vi "01 Dryer_Performance_SM.vi"() -> ()   [LabVIEW 2012] (continued)
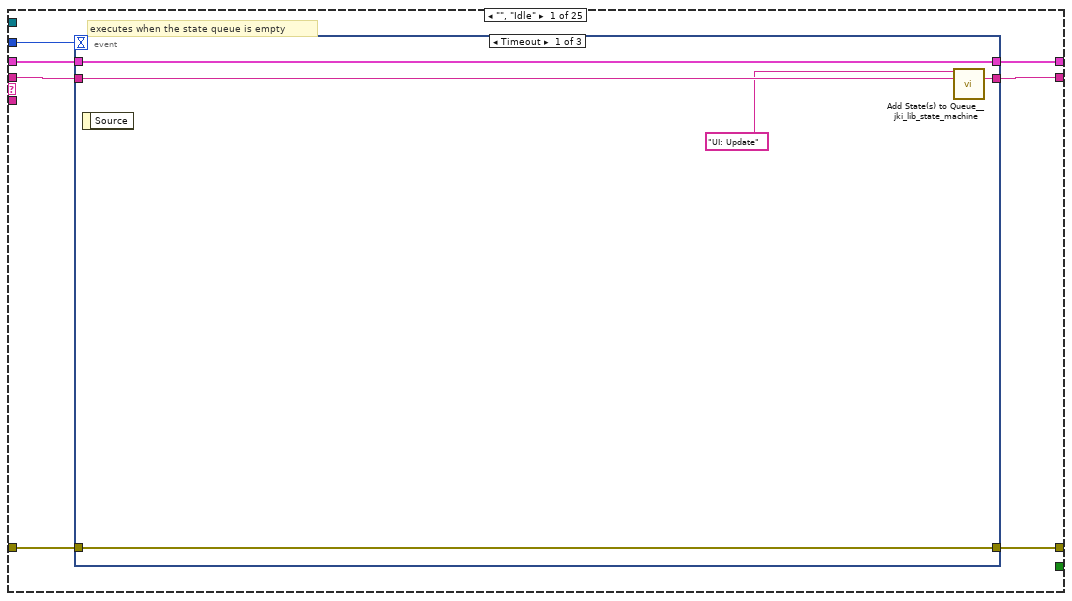
[diagram p3: hidden frame]
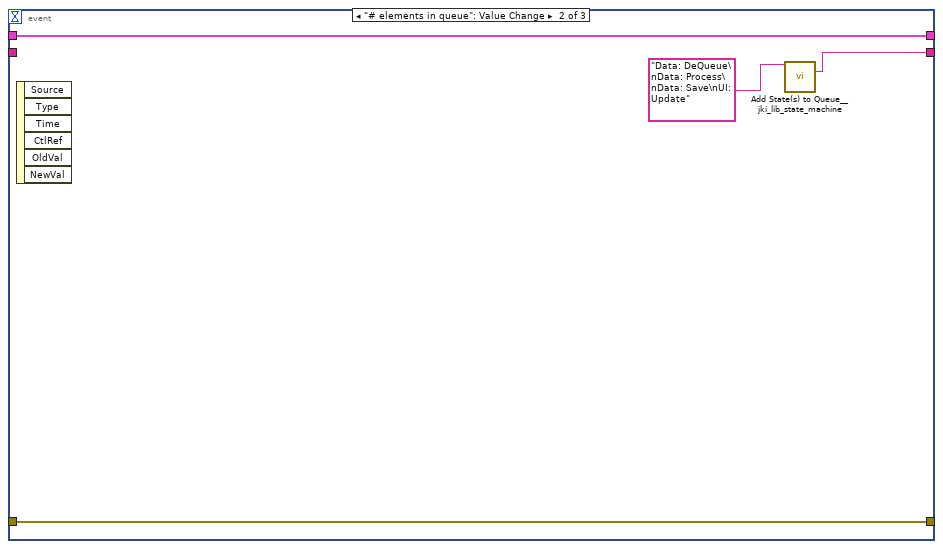
[diagram p4: hidden frame]
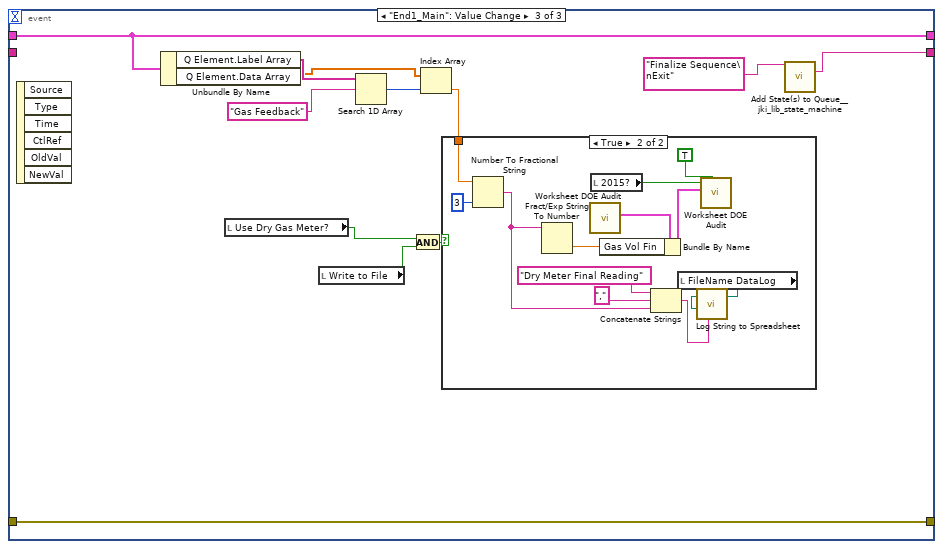
[diagram p5: hidden frame]
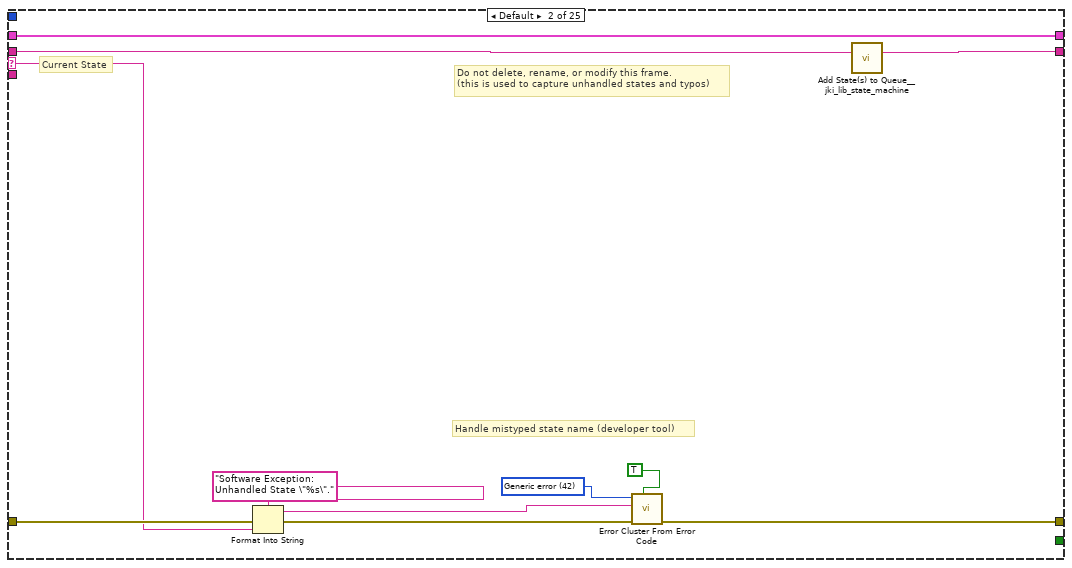
[diagram p7: hidden frame]
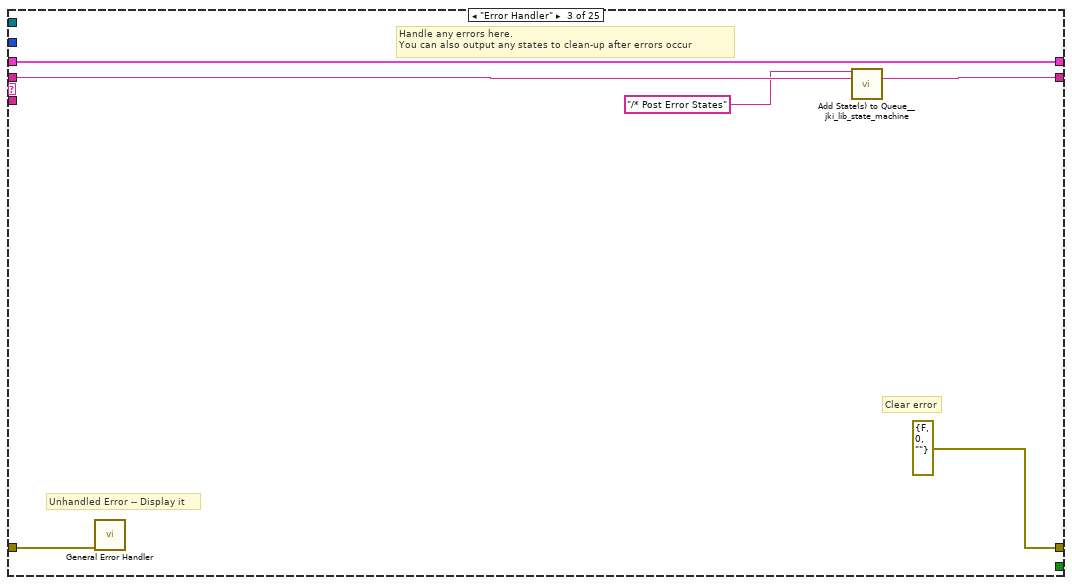
[diagram p8: hidden frame]
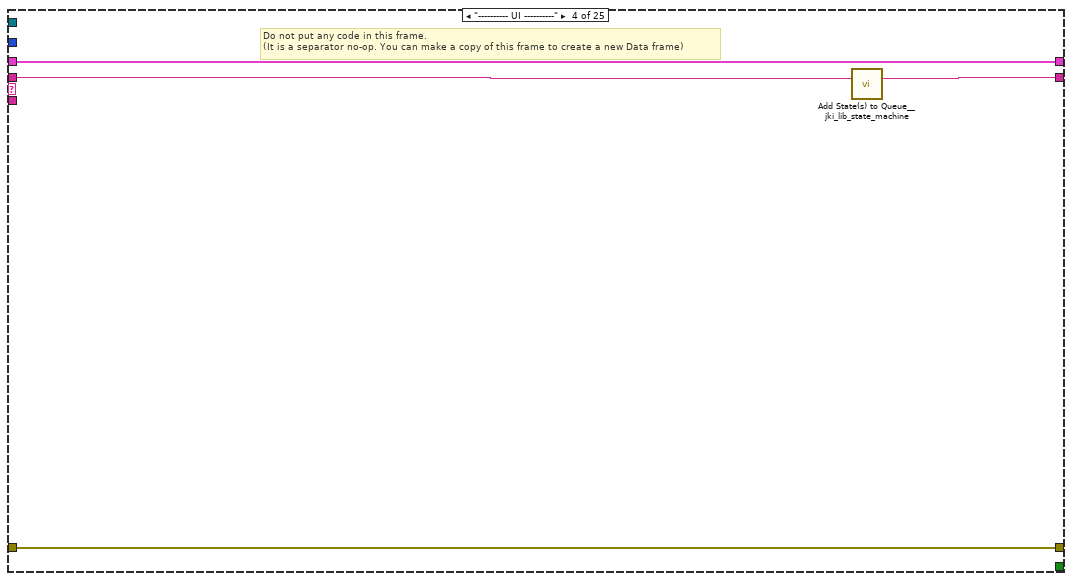
[diagram p9: hidden frame]
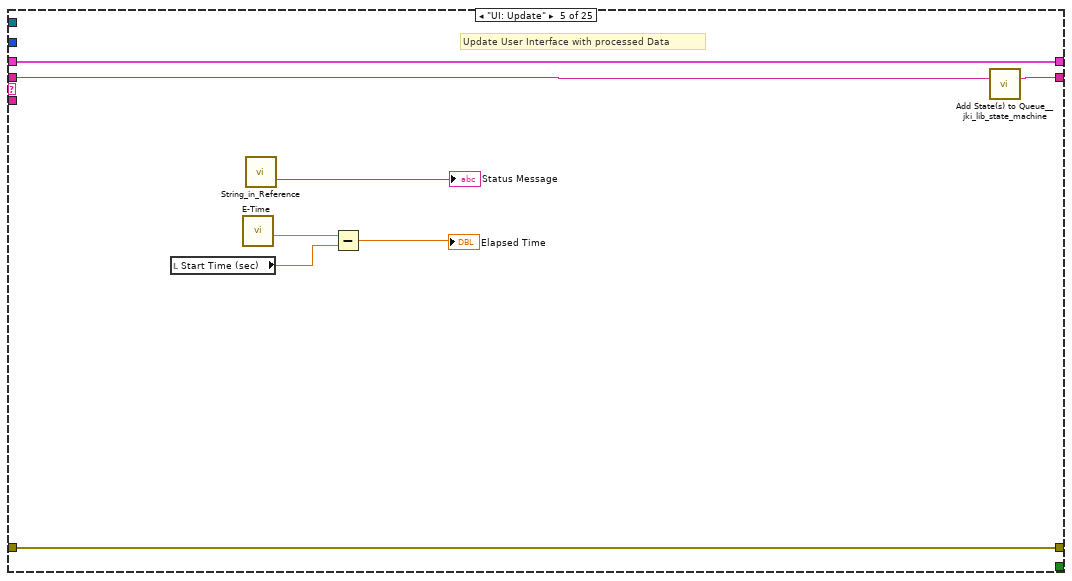
[diagram p10: hidden frame]
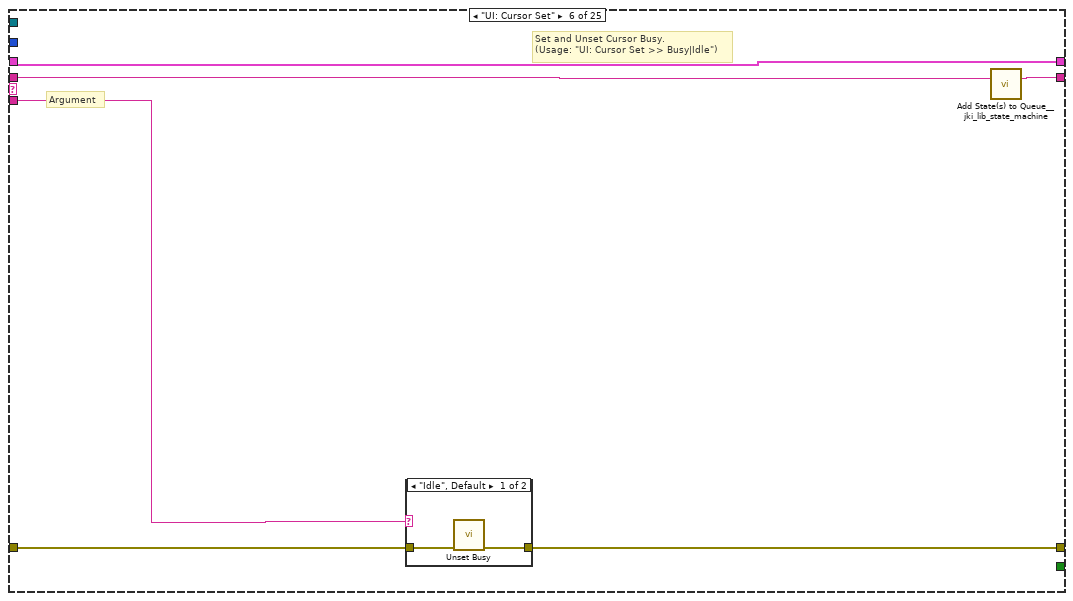
[diagram p11: hidden frame]
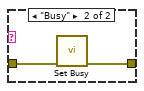
[diagram p12: hidden frame]
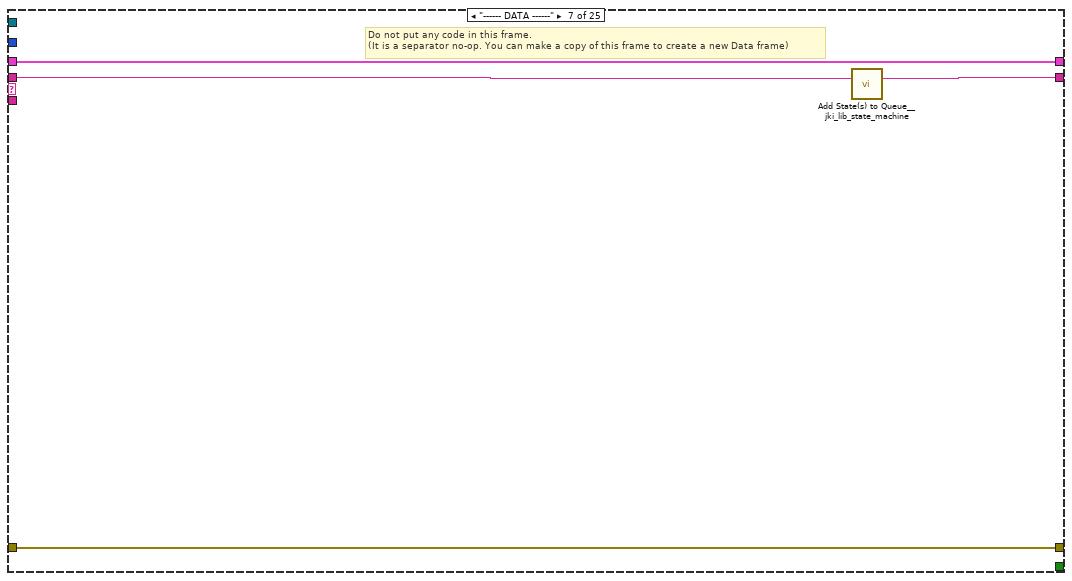
[diagram p13: hidden frame]
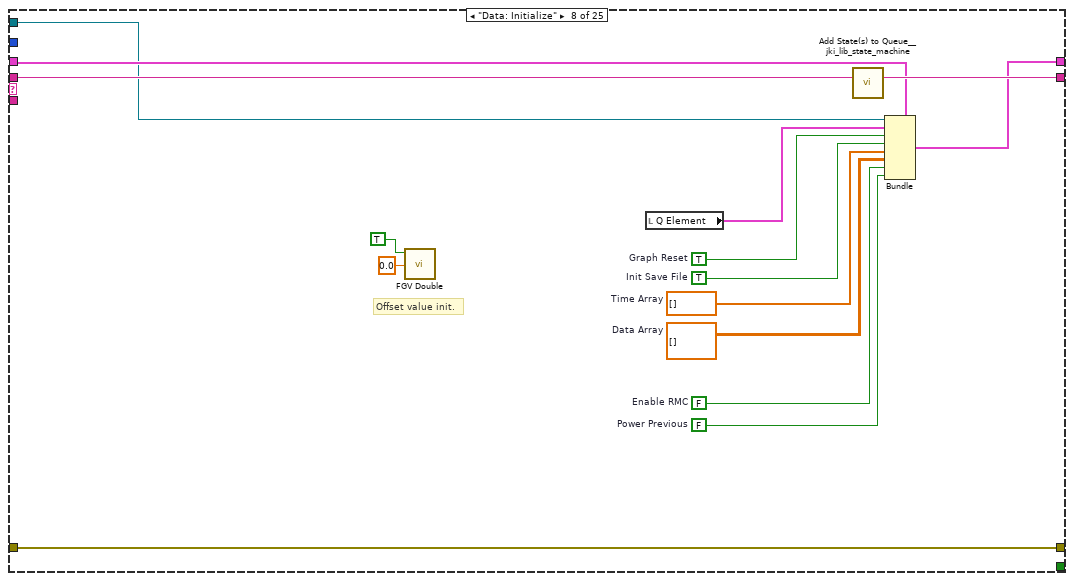
[diagram p14: hidden frame]
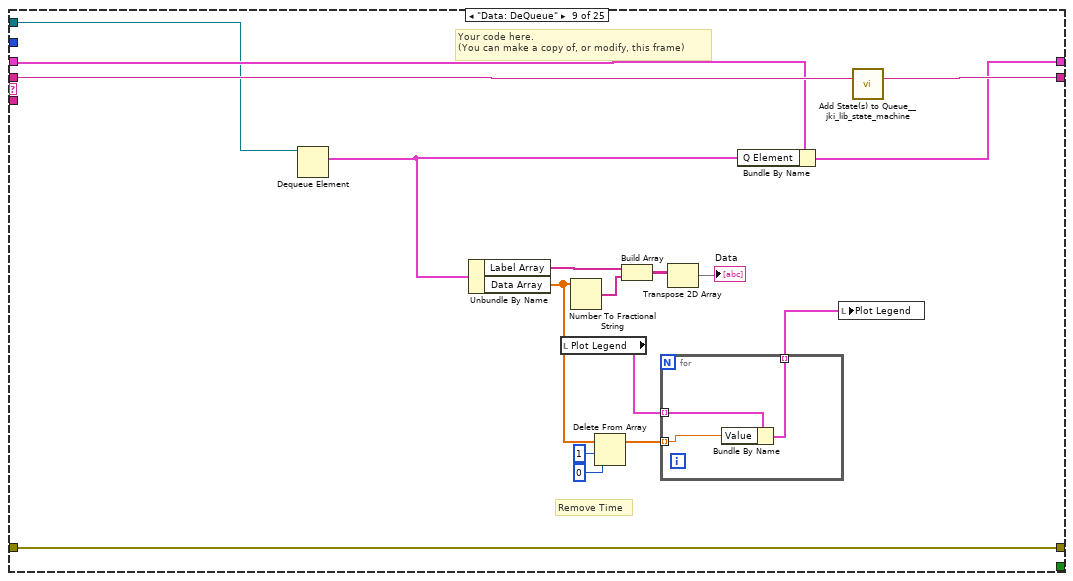
[diagram p15: hidden frame]
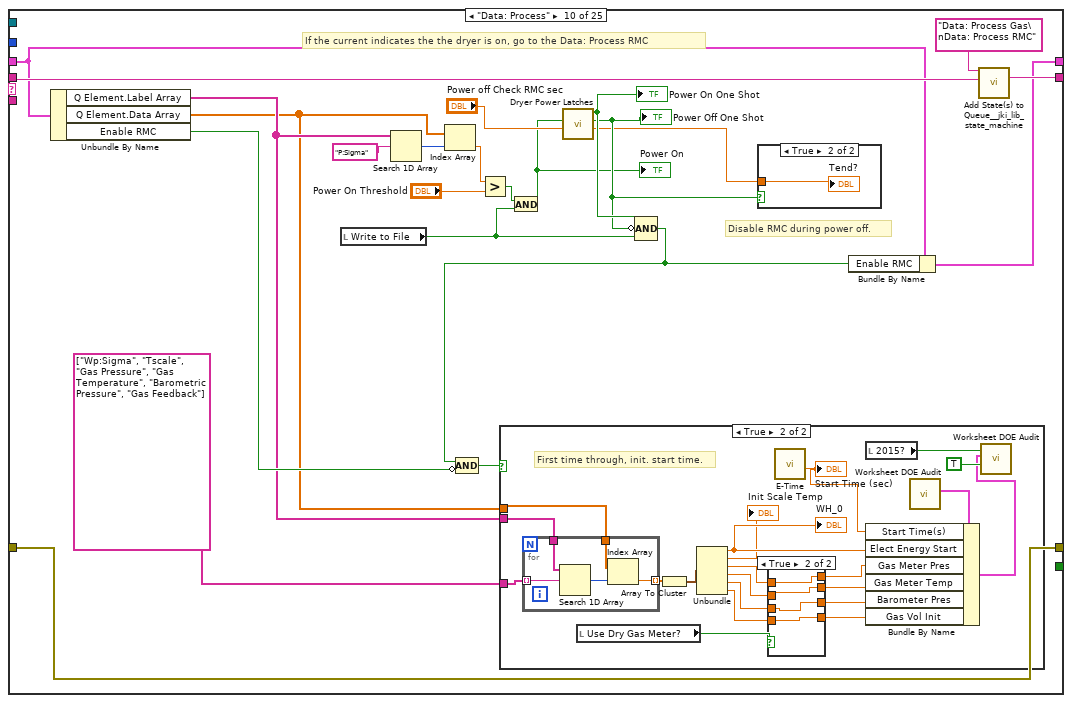
[diagram p16: hidden frame]
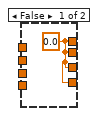
[diagram p19: hidden frame]
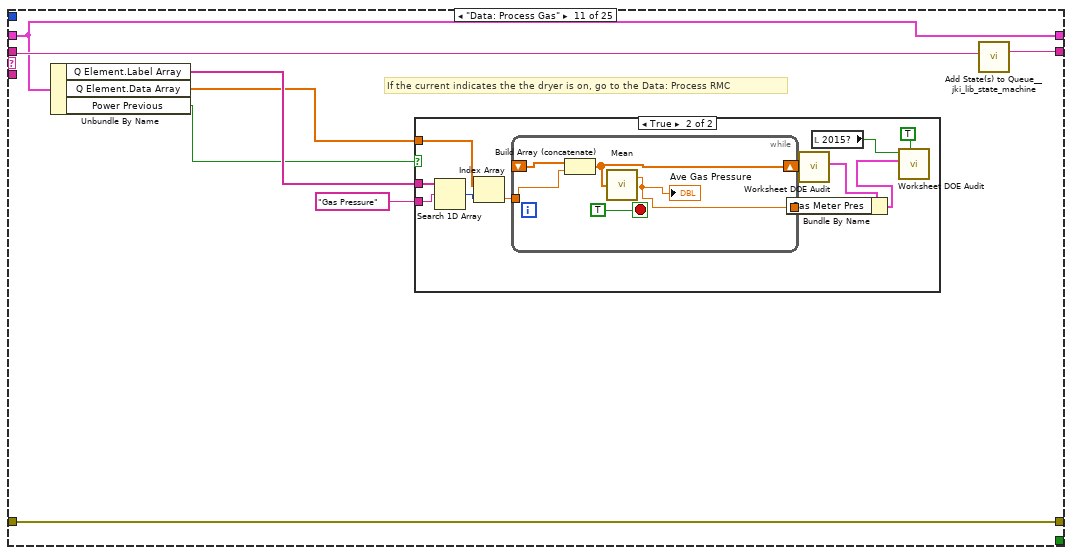
[diagram p20: hidden frame]
          }
          frame True {
            n1123 = Array Size(array=w2358) -> (size(s)=w2357:i32)
            n1124 = for {
              N: w2357 -> [_]
              tunnel: [w2361] -> w2356 mode=indexing
              n1125 = Random Number (0-1)() -> (number: 0 to 1=w2363:dbl)
              n1126 = Add(x=75.0, y=w2363) -> (x+y=w2361:dbl)
            }
          }
        }
        "Agilent Error Message" <- w2332
        "DAQ Data" <- w2323
        n1127 = Build Array (concatenate)(w2324, w2323) -> (w2326:dbl[])
        n1128 = Build Array (concatenate)(w2325, w2318) -> (w2327:string[])
        n1129 = Bundle By Name(cluster=w2334, "Q Element.Label Array"=w2327, "Q Element.Data Array"=w2326) -> (w2336:T34)
        n1130 = In Range and Coerce(upper limit=2000.0, x=w2323, lower limit=-inf) -> (In Range?=w2321:bool[])  [unwired: 1 out]
        n1131 = And Array Elements(Boolean array=w2321) -> (logical AND=w2320:bool)
        n1132 = case shown="Error" w2329 {
          tunnel: w2328 -> [_ w2343]
          frame No Error {
          }
          frame Error {
            n1133 = Concatenate Strings("Error:", w2343) -> (w2345:string)
            n1134 = One Button Dialog(message=w2345) -> ()  [unwired: 1 in, 1 out]
          }
        }
        n1135 = disable-structure shown="Disabled" {
          disable-tunnel: w2320 -> [w2339 w2342]
          frame Disabled {
            n1136 = case shown="False" w2339 {
              frame False {
                n1137 = One Button Dialog(message="Temp OOR") -> (true=w2340:bool)  [unwired: 1 in]
                n1138 = Stop(stop? (T)=w2340) -> ()
              }
              frame True {
              }
            }
          }
          frame Enabled {
            n1139 = local write "Temp OOR"(w2342) -> ()
          }
        }
        n1140 = call <vilib>:"Add State(s) to Queue__jki_lib_state_machine.vi"("State(s) in (\"\")"=w2331) -> ("States Out"=w2338:string)  [unwired: 14 in]
      }
      frame "Data Acquire: Ag + W" {
        # "First one begins array."
        # "Acquire Data Step.\n(This is an example that simulates the gathering of data.)"
        n1141 = Unbundle By Name(w2384) -> ("Q Element.Label Array"=w2376:string[], "Q Element.Data Array"=w2375:dbl[], "Equipment.Com Agilent"=w2366:refnum<visa-resource-name>)
        n1142 = local read "Simulate"() -> (w2382:bool)
        n1143 = local read "DAQ Label List"() -> (w2379:string[])
        n1144 = Equal?(x=w2366, y=refnum<visa-resource-name> "AGILENT-34980A" ("VISA resource name")) -> (x = y?=w2364:bool)
        n1145 = case shown="False" w2382 {
          tunnel: w2385 -> [w2393 w2445]
          tunnel: w2366 -> [w2394 _]
          tunnel: [w2397 w2441] -> w2368
          tunnel: [w2398 "Simulation" ("Error Message")] -> w2369
          tunnel: [w2396 w2445] -> w2381
          tunnel: w2379 -> [_ w2443]
          tunnel: [w2395 w2439] -> w2367
          tunnel: w2364 -> [w2392 _]
          frame False {
            n1146 = case shown="False" w2392 {
              tunnel: [w2412 w2421] -> w2398
              tunnel: [w2407 w2431] -> w2397
              tunnel: [w2403 w2428] -> w2396
              tunnel: [w2402 w2425] -> w2395
              tunnel: w2394 -> [w2400 w2427]
              tunnel: w2393 -> [w2399 w2426]
              frame True {
                n1147 = local read "Weight Offset"() -> (w2410:dbl)
                n1148 = local read "W.Samps"() -> (w2409:i32)
                n1149 = call "AG34980A Initiate.vi"("VISA resource name"=w2400, "error in (no error)"=w2399) -> ("VISA resource name out"=w2414:refnum<visa-resource-name>, "error out"=w2416:errorcluster)  [unwired: 12 in]
                n1150 = call "AG34980A Fetch.vi"("VISA resource name"=w2414, "Numbers Only (T:On)"=TRUE, "error in (no error)"=w2416, "Byte Count (1024 bytes)"=50000) -> ("VISA resource name out"=w2413:refnum<visa-resource-name>, "Output Data (Numbers Only)"=w2402:dbl[], "error out"=w2415:errorcluster)  [unwired: 7 in, 2 out]
                n1151 = for {
                  N: w2409 -> [_]
                  tunnel: w2410 -> [w2418]
                  tunnel: [w2417] -> w2408 mode=indexing
                  shift-right: [w2419] -> w2405
                  shift-left: w2399 -> [w2420]
                  n1152 = call "Weight Input.vi"("Offset"=w2418, "Error In"=w2420) -> ("Weight"=w2417:dbl, "error out"=w2419:errorcluster)  [unwired: 9 in, 3 out]
                }
                n1153 = call "AG34980A Error Query (Multiple).vi"("VISA resource name"=w2413, "error in (no error)"=w2415) -> ("Error Message"=w2412:string, "error out"=w2404:errorcluster)  [unwired: 10 in, 2 out]
                n1154 = call-poly <vilib>:"Mean.vi"("X"=w2408) -> ("mean"=w2406:dbl)  [unwired: 1 out]
                n1155 = Build Array (concatenate)(w2402, w2406) -> (w2407:dbl[])
                n1156 = Merge Errors(w2404, w2405) -> (w2403:errorcluster)
              }
              frame False {
                n1157 = local read "Weight Offset"() -> (w2434:dbl)
                n1158 = local read "W.Samps"() -> (w2433:i32)
                n1159 = call "Read Chans in Scan List.vi"("error in (no error)"=w2426, "VISA Resource Name"=w2427) -> ("error out"=w2423:errorcluster, "Values Array"=w2425:dbl[], "VISA Resource Name Out"=w2422:refnum<visa-resource-name>)  [unwired: 7 in]
                n1160 = for {
                  N: w2433 -> [_]
                  tunnel: w2434 -> [w2436]
                  tunnel: [w2435] -> w2432 mode=indexing
                  shift-right: [w2437] -> w2429
                  shift-left: w2426 -> [w2438]
                  n1161 = call "Weight Input.vi"("Offset"=w2436, "Error In"=w2438) -> ("Weight"=w2435:dbl, "error out"=w2437:errorcluster)  [unwired: 9 in, 3 out]
                }
                n1162 = call "Error Query (Multiple).vi"("VISA Resource Name"=w2422, "error in (no error)"=w2423) -> ("Error Message"=w2421:string, "error out"=w2424:errorcluster)  [unwired: 10 in, 2 out]
                n1163 = call-poly <vilib>:"Mean.vi"("X"=w2432) -> ("mean"=w2430:dbl)  [unwired: 1 out]
                n1164 = Build Array (concatenate)(w2425, w2430) -> (w2431:dbl[])
                n1165 = Merge Errors(w2424, w2429) -> (w2428:errorcluster)
              }
            }
          }
          frame True {
            n1166 = Array Size(array=w2443) -> (size(s)=w2442:i32)
            n1167 = for {
              N: w2442 -> [_]
              tunnel: [w2446] -> w2439 mode=indexing
              n1168 = Random Number (0-1)() -> (number: 0 to 1=w2448:dbl)
              n1169 = Add(x=75.0, y=w2448) -> (x+y=w2446:dbl)
            }
            n1170 = Build Array (concatenate)(w2439, 100.0 ("Mean")) -> (w2441:dbl[])
          }
        }
        n1171 = Build Array (concatenate)(w2376, w2379, string[] ["Weight"] ("element")) -> (w2378:string[])
        n1172 = Build Array (concatenate)(w2375, w2368) -> (w2377:dbl[])
        n1173 = Bundle By Name(cluster=w2384, "Q Element.Label Array"=w2378, "Q Element.Data Array"=w2377) -> (w2386:T34)
        n1174 = local write "DAQ Data"(w2367) -> ()
        n1175 = local write "Agilent Error Message"(w2369) -> ()
        n1176 = case shown="Error" w2381 {
          tunnel: w2380 -> [_ w2389]
          frame No Error {
          }
          frame Error {
            n1177 = Concatenate Strings("Error:", w2389) -> (w2391:string)
            n1178 = One Button Dialog(message=w2391) -> ()  [unwired: 1 in, 1 out]
          }
        }
        n1179 = In Range and Coerce(upper limit=2000.0, x=w2368, lower limit=-inf) -> (In Range?=w2372:bool[])  [unwired: 1 out]
        "In Range?" <- w2372
        n1180 = And Array Elements(Boolean array=w2372) -> (logical AND=→"Temp OOR":bool)
        n1181 = call <vilib>:"Add State(s) to Queue__jki_lib_state_machine.vi"("State(s) in (\"\")"=w2383) -> ("States Out"=w2388:string)  [unwired: 14 in]
      }
      frame "Data Acquire: CDAQ" {
        # "First one begins array."
        # "Acquire Data Step.\n(This is an example that simulates the gathering of data.)"
        n1182 = Unbundle By Name(w2471) -> ("Q Element.Label Array"=w2462:string[], "Q Element.Data Array"=w2461:dbl[], "Equipment.Com Agilent"=w2470:refnum<visa-resource-name>, "DAQ Chanel List"=w2452:string)
        n1183 = local read "DAQ Label List"() -> (w2465:string[])
        n1184 = local read "Simulate"() -> (w2468:bool)
        n1185 = Spreadsheet String To Array(delimiter (Tab)=",", format string="", spreadsheet string=w2452, array type (2D Dbl)=i32[] []) -> (array=w2451:i32[])
        n1186 = case shown="False" w2468 {
          tunnel: w2472 -> [w2498 w2517]
          tunnel: w2470 -> [_ _]
          tunnel: [w2501 w2514] -> w2456
          tunnel: [w2499 w2517] -> w2467
          tunnel: w2465 -> [_ w2516]
          tunnel: [w2494 w2512] -> w2455
          tunnel: w2451 -> [w2495 _]
          frame False {
            n1187 = local read "Write to File"() -> (w2488:bool)
            n1188 = local read "Stream DC to File?"() -> (w2490:bool)
            n1189 = local read "Weight Offset"() -> (w2504:dbl)
            n1190 = local read "W.Samps"() -> (w2503:i32)
            n1191 = And(x=w2488, y=w2490) -> (x .and. y?=w2489:bool)
            n1192 = local read "CDAQ Tasks"() -> (w2492:refnum<k21>[])
            n1193 = call "03 cDAQ Chan Tester.vi"("Tasks In"=w2492, "error in (no error)"=w2498, "Stream Voltages to File"=w2489, "DC Voltages Filename"="DC Voltages Filename", "Mode"=T18."Gather DATA") -> ("error out"=w2497:errorcluster, "CDAQ Data Out"=w2494:dbl[])  [unwired: 4 in, 1 out]
            n1194 = for {
              N: w2503 -> [_]
              tunnel: w2504 -> [w2509]
              tunnel: [w2508] -> w2502 mode=indexing
              shift-right: [w2510] -> w2487
              shift-left: w2498 -> [w2511]
              n1195 = call "Weight Input.vi"("Offset"=w2509, "Error In"=w2511) -> ("Weight"=w2508:dbl, "error out"=w2510:errorcluster)  [unwired: 9 in, 3 out]
            }
            n1196 = for {
              tunnel: [w2506] -> w2496 mode=indexing
              tunnel: w2494 -> [w2507]
              tunnel: w2495 -> [w2505] mode=indexing
              n1197 = Index Array(array=w2507, index=w2505) -> (element=w2506:dbl)
            }
            n1198 = call "Door Switch.vi"("error in (no error)"=w2487) -> ("error out"=w2486:errorcluster, "Door Switch Activation"=w2485:i16)  [unwired: 9 in]
            n1199 = call-poly <vilib>:"Mean.vi"("X"=w2502) -> ("mean"=w2500:dbl)  [unwired: 1 out]
            n1200 = Build Array (concatenate)(w2496, w2500, w2485) -> (w2501:dbl[])
            n1201 = Merge Errors(w2497, w2486) -> (w2499:errorcluster)
          }
          frame True {
            n1202 = Array Size(array=w2516) -> (size(s)=w2515:i32)
            n1203 = for {
              N: w2515 -> [_]
              tunnel: [w2518] -> w2512 mode=indexing
              n1204 = Random Number (0-1)() -> (number: 0 to 1=w2520:dbl)
              n1205 = Add(x=75.0, y=w2520) -> (x+y=w2518:dbl)
            }
            n1206 = Build Array (concatenate)(w2512, 100.0 ("Mean")) -> (w2514:dbl[])
          }
        }
        n1207 = Build Array (concatenate)(w2462, w2465, string[] ["Weight", "Door Switch"] ("element")) -> (w2464:string[])
        n1208 = Build Array (concatenate)(w2461, w2456) -> (w2463:dbl[])
        n1209 = Bundle By Name(cluster=w2471, "Q Element.Label Array"=w2464, "Q Element.Data Array"=w2463) -> (w2473:T34)
        n1210 = local write "DAQ Data"(w2455) -> ()
        n1211 = In Range and Coerce(upper limit=2000.0, x=w2456, lower limit=-inf) -> (In Range?=w2454:bool[])  [unwired: 1 out]
        n1212 = And Array Elements(Boolean array=w2454) -> (logical AND=w2458:bool)
        n1213 = case shown="Error" w2467 {
          tunnel: w2466 -> [_ w2482]
          frame No Error {
          }
          frame Error {
            n1214 = Concatenate Strings("Error:", w2482) -> (w2484:string)
            n1215 = Two Button Dialog(message=w2484, 2:"Stop" ("T button name (\"OK\")")) -> (T button?=w2480:bool)  [unwired: 1 in]
            n1216 = case shown="True" w2480 {
              frame False {
              }
              frame True {
                n1217 = Stop() -> ()  [unwired: 1 in]
              }
            }
          }
        }
        n1218 = disable-structure shown="Enabled" {
          disable-tunnel: w2458 -> [w2476 w2479]
          frame Disabled {
            n1219 = case shown="False" w2476 {
              frame False {
                n1220 = One Button Dialog(message="Temp OOR") -> (true=w2477:bool)  [unwired: 1 in]
                n1221 = Stop(stop? (T)=w2477) -> ()
              }
              frame True {
              }
            }
          }
          frame Enabled {
            n1222 = local write "Temp OOR"(w2479) -> ()
          }
        }
        n1223 = local write "In Range?"(w2454) -> ()
        n1224 = call <vilib>:"Add State(s) to Queue__jki_lib_state_machine.vi"("State(s) in (\"\")"=w2469) -> ("States Out"=w2475:string)  [unwired: 14 in]
      }
      frame "Data Acquire: Power" {
        (unwired) string[] ["VL1", "VL2", "IL1", "IL2", "P", "WH", "Ipeak", "Phi(1,2)"]
        # "Acquire Data Step.\n(This is an example that simulates the gathering of data.)"
        n1225 = Unbundle By Name(w2534) -> ("Q Element.Label Array"=w2529:string[], "Q Element.Data Array"=w2533:dbl[], "Equipment.Com Power Meter"=w2531:refnum<visa-resource-name>)  [unwired: 1 out]
        n1226 = local read "Power Label"() -> (w2523:string[])
        n1227 = local read "Simulate"() -> (w2526:bool)
        n1228 = case shown="False" w2526 {
          tunnel: [w2545 T3 {"Current L1"=236.2, "Current L2"=17.749, "Power"=4192.0, "WattHours"=0.0} ("PowerData")] -> w2522
          tunnel: w2531 -> [w2544 _]
          tunnel: w2530 -> [w2542 w2551]
          tunnel: [w2541 w2551] -> w2521
          tunnel: [w2540 w2548] -> w2525
          tunnel: w2523 -> [_ w2546]
          tunnel: [w2539 w2546] -> w2524
          frame False {
            n1229 = call "WT500 Read Power.vi"("VISA resource name"=w2544, "WT500 CMDS"=WT500_Sequences."GetReadings", "error in (no error)"=w2542) -> ("PowerData"=w2545:T3, "Measurement Values"=w2540:dbl[], "Label"=w2539:string[], "error out"=w2541:errorcluster)  [unwired: 7 in, 2 out]
          }
          frame True {
            n1230 = Array Size(array=w2546) -> (size(s)=w2549:i32)
            n1231 = Initialize Array(0.0 ("element"), w2549) -> (w2548:dbl[])
          }
        }
        "PowerData" <- w2522
        n1232 = Build Array (concatenate)(w2529, w2524) -> (w2528:string[])
        n1233 = Build Array (concatenate)(w2533, w2525) -> (w2532:dbl[])
        n1234 = case shown="Error" w2521 {
          tunnel: w2527 -> [_ w2552]
          frame No Error {
          }
          frame Error {
            n1235 = One Button Dialog(message=w2552) -> ()  [unwired: 1 in, 1 out]
          }
        }
        n1236 = Bundle By Name(cluster=w2534, "Q Element.Label Array"=w2528, "Q Element.Data Array"=w2532) -> (w2535:T34)
        n1237 = call <vilib>:"Add State(s) to Queue__jki_lib_state_machine.vi"("State(s) in (\"\")"=w2538) -> ("States Out"=w2537:string)  [unwired: 14 in]
      }
      frame "Data Acquire: Gas" {
        # "FIXME: VERIFY CORRECT READINGS."
        # "Acquire Data Step.\n(This is an example that simulates the gathering of data.)"
        n1238 = Unbundle By Name(w2567) -> ("Q Element.Label Array"=w2564:string[], "Q Element.Data Array"=w2566:dbl[], "Equipment.Com Flow Computer"=w2561:refnum<visa-resource-name>)
        n1239 = local read "Simulate"() -> (w2553:bool)
        n1240 = Or(x=w2553, y=TRUE) -> (x .or. y?=w2554:bool)
        n1241 = case shown="False" w2554 {
          tunnel: w2560 -> [w2577 w2580]
          tunnel: [w2576 w2580] -> w2559
          tunnel: w2561 -> [w2572 _]
          tunnel: [w2575 string[] [] ("array")] -> w2557
          tunnel: [w2574 string[] [] ("array")] -> w2558
          frame False {
            n1242 = local read "Use SL9200 Gas Readings?"() -> (w2579:bool)
            n1243 = local read "Use Dry Gas Meter?"() -> (w2578:bool)
            n1244 = call "Gas Flow Readings.vi"("Com Flow Computer"=w2572, "Use SL9200 Gas Readings?"=w2579, "Use Dry Gas Meter?"=w2578, "Initialize?"=FALSE, "Error In"=w2577) -> ("Labels"=w2574:string[], "Values"=w2575:string[], "error out"=w2576:errorcluster)  [unwired: 8 in]
          }
          frame True {
            # "Not reading encoder\nanymore!"
          }
        }
        n1245 = Build Array (concatenate)(w2564, w2558) -> (w2563:string[])
        n1246 = Fract/Exp String To Number(string=w2557) -> (number=w2556:dbl[])  [unwired: 3 in, 1 out]
        n1247 = Build Array (concatenate)(w2566, w2556) -> (w2565:dbl[])
        n1248 = Bundle By Name(cluster=w2567, "Q Element.Label Array"=w2563, "Q Element.Data Array"=w2565) -> (w2568:T34)
        n1249 = case shown="Error" w2559 {
          tunnel: w2562 -> [_ w2583]
          frame No Error {
          }
          frame Error {
            n1250 = One Button Dialog(message=w2583) -> ()  [unwired: 1 in, 1 out]
          }
        }
        n1251 = call <vilib>:"Add State(s) to Queue__jki_lib_state_machine.vi"("State(s) in (\"\")"=w2571) -> ("States Out"=w2570:string)  [unwired: 14 in]
      }
      frame "Data Acquire: RH" {
        # "Acquire Data Step.\nAcquire data from ITHX logger if values of IP are not 0.  This should be set in the global config.\nGet RH vals.  First time thru loop, look for headers and replace values.  Otherwise, concatonate values."
        n1252 = global read "Global Test Variables DPT.vi" "Globals for Dryer Performance Test"() -> (w2593:T9)
        n1253 = Unbundle By Name(w2597) -> ("Q Element.Label Array"=w2588:string[], "Q Element.Data Array"=w2587:dbl[])
        n1254 = Unbundle By Name(w2593) -> ("Test Setup.RH-IP"=w2592:string, "Test Setup.RH-IP2"=w2591:string, "Test Setup.RH-IP3"=w2590:string)
        n1255 = Build Array(w2592, w2591, w2590) -> (w2589:string[])
        n1256 = for {
          tunnel: w2595 -> [w2612]
          tunnel: [w2611] -> w2594
          tunnel: w2589 -> [w2603] mode=indexing
          shift-right: [w2608] -> w2586
          shift-left: w2588 -> [w2607]
          shift-right: [w2606] -> w2585
          shift-left: w2587 -> [w2605]
          tunnel: string[][] [["Chamber Temp", "Chamber RH"], ["Probe1 Temp", "Probe1 RH"], ["Probe2 Temp", "Probe2 RH"]] ("array") -> [w2602] mode=indexing
          i -> [w2604]
          # "FIXME: VERIFY CORRECT READINGS."
          n1257 = Equal?(x=w2603, y="0") -> (x = y?=w2610:bool)
          n1258 = case shown="False" w2610 {
            tunnel: w2612 -> [w2619 w2644]
            tunnel: [w2620 w2644] -> w2611
            tunnel: [w2613 w2643] -> w2608
            tunnel: w2607 -> [w2617 w2643]
            tunnel: [w2614 w2642] -> w2606
            tunnel: w2605 -> [w2615 w2642]
            tunnel: w2604 -> [w2623 _]
            tunnel: w2603 -> [w2621 _]
            tunnel: w2602 -> [w2616 _]
            frame False {
              n1259 = Equal To 0?(x=w2623) -> (x = 0?=w2622:bool)
              n1260 = call "Newport ITX-D3N.vi"("error in (no error)"=w2619, "Machine"=w2621) -> ("error out"=w2620:errorcluster, "[Temp (F), RH]"=w2618:dbl[])  [unwired: 8 in]
              "[Temp (F), RH]" <- w2618
              n1261 = case shown="True" w2622 {
                tunnel: w2618 -> [w2624 w2635]
                tunnel: w2617 -> [w2628 w2634]
                tunnel: w2616 -> [w2627 w2633]
                tunnel: w2615 -> [w2626 w2632]
                tunnel: [w2625 w2631] -> w2614
                tunnel: [w2629 w2630] -> w2613
                frame False {
                  n1262 = Build Array (concatenate)(w2626, w2624) -> (w2625:dbl[])
                  n1263 = Build Array (concatenate)(w2628, w2627) -> (w2629:string[])
                }
                frame True {
                  n1264 = for {
                    tunnel: w2635 -> [w2641] mode=indexing
                    tunnel: w2634 -> [w2637]
                    tunnel: w2633 -> [w2640] mode=indexing
                    shift-right: [w2638] -> w2631
                    shift-left: w2632 -> [w2639]
                    tunnel: [w2637] -> w2630
                    n1265 = Search 1D Array(1D array=w2637, element=w2640) -> (index of element=w2636:i32)  [unwired: 1 in]
                    n1266 = Replace Array Subset(array=w2639, new element=w2641, index=w2636) -> (w2638:dbl[])
                  }
                }
              }
            }
            frame True {
              # "If the IP is configured, replace the Chamber RH\nand Temp with Ithx values.\nIf second and 3rd configured, add them."
            }
          }
        }
        n1267 = Bundle By Name(cluster=w2597, "Q Element.Label Array"=w2586, "Q Element.Data Array"=w2585) -> (w2598:T34)
        n1268 = case shown="Error" w2594 {
          tunnel: w2596 -> [_ w2645]
          frame No Error {
          }
          frame Error {
            n1269 = One Button Dialog(message=w2645) -> ()  [unwired: 1 in, 1 out]
          }
        }
        n1270 = call <vilib>:"Add State(s) to Queue__jki_lib_state_machine.vi"("State(s) in (\"\")"=w2601) -> ("States Out"=w2600:string)  [unwired: 14 in]
      }
      frame "Data Acquire: Weight" {
        # "acquire weight.  take 5 samples and averge"
        n1271 = case shown="True" "USB Weight?" {
          tunnel: [w2654 w2666] -> w2650
          tunnel: w2649 -> [w2654 w2665]
          tunnel: w2648 -> [w2655 w2664]
          tunnel: [w2655 w2663] -> w2647
          frame False {
          }
          frame True {
            n1272 = Unbundle By Name(w2665) -> ("Q Element.Label Array"=w2659:string[], "Q Element.Data Array"=w2661:dbl[])
            n1273 = local read "Simulate"() -> (w2656:bool)
            n1274 = case shown="False" w2656 {
              tunnel: w2664 -> [w2672 w2678]
              tunnel: [w2671 w2678] -> w2663
              tunnel: [w2667 100.0 ("Mean")] -> w2662
              frame False {
                n1275 = for {
                  N: "W.Samps" -> [_]
                  tunnel: "Weight Offset" -> [w2674]
                  tunnel: [w2673] -> w2668 mode=indexing
                  shift-right: [w2675] -> w2671
                  shift-left: w2672 -> [w2676]
                  n1276 = call "Weight Input.vi"("Offset"=w2674, "Error In"=w2676) -> ("Weight"=w2673:dbl, "error out"=w2675:errorcluster)  [unwired: 9 in, 3 out]
                }
                n1277 = call-poly <vilib>:"Mean.vi"("X"=w2668) -> ("mean"=w2667:dbl)  [unwired: 1 out]
              }
              frame True {
              }
            }
            n1278 = Build Array (concatenate)(w2659, string[] ["Weight"] ("element")) -> (w2657:string[])
            n1279 = Build Array (concatenate)(w2661, w2662) -> (w2660:dbl[])
            n1280 = Bundle By Name(cluster=w2665, "Q Element.Label Array"=w2657, "Q Element.Data Array"=w2660) -> (w2666:T34)
          }
        }
        n1281 = call <vilib>:"Add State(s) to Queue__jki_lib_state_machine.vi"("State(s) in (\"\")"=w2653) -> ("States Out"=w2652:string)  [unwired: 14 in]
      }
      frame "Data: Queue" {
        # "Put Data in Queue to be used by parsing/saving code ->"
        n1282 = Unbundle By Name(w2681) -> ("Q Element"=w2680:T10)  [unwired: 1 out]
        n1283 = Enqueue Element(queue=w2679, element=w2680) -> (queue out=w2684:refnum<queue>)  [unwired: 2 in, 2 out]
        n1284 = Get Queue Status(queue=w2684) -> (# elements in queue=w2683:i32)  [unwired: 2 in, 7 out]
        "# elements in queue" <- w2683
        n1285 = property on="# elements in queue" class="DigNum (strict)"("Val(Sgnl)"=w2683) -> ()  [unwired: 2 in, 2 out]
        n1286 = call <vilib>:"Add State(s) to Queue__jki_lib_state_machine.vi"("State(s) in (\"\")"=w2687) -> ("States Out"=w2686:string)  [unwired: 14 in]
      }
    }
    n1287 = local read "Debug Mode"() -> (w2195:bool)
    n1288 = case shown="True" w2195 {
      tunnel: [w2209 w2212] -> w2198
      tunnel: w2197 -> [w2209 w2211]
      tunnel: w2196 -> [_ w2210]
      frame False {
      }
      frame True {
        n1289 = Build Array (concatenate)(w2211, w2210) -> (w2212:string[])
        "daq debug array" <- w2212
      }
    }
  }
  n1290 = event shown="[0] \"stop\": Value Change" {
    selector: _ -> [_ _]
    dyn-events: _ -> [_ _]
    timeout: _ -> [_ _]
    tunnel: [FALSE ("stop") FALSE ("stop")] -> w5
    event "stop": Value Change {
      w2688 = TRUE ("Exit Nufi")
      n1291 = event-data() -> ()  [unwired: 1 in, 3 out]
      n1292 = while {
        stop <- w2695 stop-if-true
        n1293 = local read "End4_Nufi"() -> (w2691:bool)
        n1294 = local read "End_End"() -> (w2690:bool)
        n1295 = local read "End2_DAQ"() -> (w2694:bool)
        n1296 = local read "Eng3_Log"() -> (w2693:bool)
        n1297 = Compound Arithmetic op=AND(w2690, w2691, w2694, w2693) -> (w2695:bool)
        n1298 = Wait (ms)(milliseconds to wait=u32 150) -> ()  [unwired: 1 out]
      }
      n1299 = global write "Nufi Global_ReceivedDataCluster.vi" "Exit Nufi"(w2688) -> ()
      n1300 = property on="End1_Main" class="Bool (strict)"("Val(Sgnl)"=w2688) -> ()  [unwired: 2 in, 2 out]
    }
    event "stop!": Value Change {
      n1301 = event-data() -> ()  [unwired: 1 in, 3 out]
      n1302 = Stop(stop? (T)="stop!") -> ()
    }
  }
  n1303 = flat-sequence {
    tunnel: w5 -> [w2698]
    frame #0 {
      n1304 = local write "stop"(w2698) -> ()
      n1305 = disable-structure shown="Enabled" {
        frame Disabled {
          n1306 = call <vilib>:"System Exec.vi"("command line"="cmd /c taskkill /F /IM \"Dryer Performance Test.exe\" ") -> ()  [unwired: 7 in, 4 out]
        }
        frame Enabled {
        }
      }
    }
  }
  n1307 = disable-structure shown="Enabled" {
    disable-tunnel: w10 -> [w2703 _]
    disable-tunnel: w9 -> [w2702 _]
    disable-tunnel: [w2701 FALSE ("End_End")] -> w20
    disable-tunnel: w7 -> [w2700 _]
    frame Enabled {
      n1308 = flat-sequence {
        tunnel: w2703 -> [_]
        tunnel: w2702 -> [_]
        tunnel: [w2705] -> w2701
        tunnel: w2700 -> [w2705]
        frame #0 {
          n1309 = local read "CDAQ Tasks"() -> (w2709:refnum<k21>[])
          n1310 = call "03 cDAQ Chan Tester.vi"("Tasks In"=w2709, "Mode"=T18."Close") -> ("error out"=w2707:errorcluster)  [unwired: 7 in, 2 out]
          n1311 = call <vilib>:"DAQmx Clear Task.vi"("task in"=refnum<k21> "Weight" ("task/channels in")) -> ("error out"=w2704:errorcluster)  [unwired: 14 in]
          n1312 = call <vilib>:"Simple Error Handler.vi"("error in (no error)"=w2707) -> ()  [unwired: 4 in, 5 out]
          n1313 = call <vilib>:"Simple Error Handler.vi"("error in (no error)"=w2704) -> ()  [unwired: 4 in, 5 out]
        }
      }
    }
    frame Disabled {
    }
  }
  "End_End" <- w20
  n1314 = flat-sequence {
    tunnel: w11 -> [w2713]
    tunnel: w21 -> [_]
    tunnel: [w2711] -> w3
    tunnel: w8 -> [w2711]
    frame #0 {
      n1315 = Release Queue(queue=w2713, force destroy? (F)=TRUE) -> ()  [unwired: 1 in, 3 out]
    }
  }
  n1316 = flat-sequence {
    tunnel: w26 -> [w2714]
    tunnel: [w2714] -> w25
    frame #0 {
      n1317 = local read "Final User Message"() -> (w2715:string)
      n1318 = One Button Dialog(message=w2715) -> ()  [unwired: 1 in, 1 out]
    }
  }
  n1319 = property on="stop" class="Bool (strict)"("Val(Sgnl)"=w20) -> ()  [unwired: 2 in, 2 out]
  "Eng3_Log" <- w25
  "End2_DAQ" <- w3
